vi "Variant Read.vi"   [LabVIEW 2021, in "Ring Buffer Strict Accessor Unit Tests.lvlib"]
uses:
  Ring Buffer Strict Accessor Unit Tests.lvlib
  <vilib>/Utility/Data Type/Type Definitions/Data Type.ctl
  Source/SubVIs/Endianess.ctl
  4dddbd7f-7a37-4b30-b909-1420f6624c69.vi
  9f68938b-e704-4d93-b96c-76448c5e5cfd.vi
  8e334985-5f37-4127-8ba8-a9867f1f09de.vi
  fedf0e91-6876-4bdd-8e42-2782282ca75b.vi
  21e74d2b-f5ac-4ba9-b347-dd9c42e89ba9.vi
  8a9216e5-439f-4ec4-b565-879cfa18150d.vi
  3161eb3e-d1dc-4e30-b8f9-f2ede20ab9bc.vi
  041afb3c-c61b-4d60-aacb-d153d2ee3189.vi
  26201e5a-6935-4402-8858-a5fc3b6697ee.vi
  4dddbd7f-7a37-4b30-b909-1420f6624c69.vi/4c2a6c61-f100-483c-8a49-51e57025a24c.vi
  4dddbd7f-7a37-4b30-b909-1420f6624c69.vi/e57bc314-87c7-4952-9bc8-929005dac297.vi
  <userlib>/bjustice/Ring Buffer for Time Series Data/API Poly.vi
  <userlib>/bjustice/Ring Buffer for Time Series Data/API/Write Array.vi
  9f68938b-e704-4d93-b96c-76448c5e5cfd.vi/f2df9050-0eef-46c6-aff6-3ce3a8893ea5.vi
  8e334985-5f37-4127-8ba8-a9867f1f09de.vi/17d75e1a-130a-47e0-8f2c-6c7d90b8ca77.vi
  <userlib>/bjustice/Ring Buffer for Time Series Data/API/Read Latest Value.vi
  Source/SubVIs/Index ByteArray.vi
  8e334985-5f37-4127-8ba8-a9867f1f09de.vi/19bdd28a-0674-4be3-87bb-ec701e431d75.vi
  Source/SubVIs/error if empty buffer.vi
  Source/SubVIs/ByteArray to Variant.vi
  fedf0e91-6876-4bdd-8e42-2782282ca75b.vi/4c2a6c61-f100-483c-8a49-51e57025a24c.vi
  fedf0e91-6876-4bdd-8e42-2782282ca75b.vi/e57bc314-87c7-4952-9bc8-929005dac297.vi
  21e74d2b-f5ac-4ba9-b347-dd9c42e89ba9.vi/f2df9050-0eef-46c6-aff6-3ce3a8893ea5.vi
  8a9216e5-439f-4ec4-b565-879cfa18150d.vi/17d75e1a-130a-47e0-8f2c-6c7d90b8ca77.vi
  8a9216e5-439f-4ec4-b565-879cfa18150d.vi/19bdd28a-0674-4be3-87bb-ec701e431d75.vi
  3161eb3e-d1dc-4e30-b8f9-f2ede20ab9bc.vi/4c2a6c61-f100-483c-8a49-51e57025a24c.vi
  3161eb3e-d1dc-4e30-b8f9-f2ede20ab9bc.vi/e57bc314-87c7-4952-9bc8-929005dac297.vi
  041afb3c-c61b-4d60-aacb-d153d2ee3189.vi/f2df9050-0eef-46c6-aff6-3ce3a8893ea5.vi
  26201e5a-6935-4402-8858-a5fc3b6697ee.vi/17d75e1a-130a-47e0-8f2c-6c7d90b8ca77.vi
  26201e5a-6935-4402-8858-a5fc3b6697ee.vi/19bdd28a-0674-4be3-87bb-ec701e431d75.vi
  <userlib>/bjustice/Ring Buffer for Time Series Data/SubVIs/Split Values Array.vi
  <userlib>/bjustice/Ring Buffer for Time Series Data/SubVIs/Replace Values Array Multiple Timestamps.vi
  9f68938b-e704-4d93-b96c-76448c5e5cfd.vi/f2df9050-0eef-46c6-aff6-3ce3a8893ea5.vi/63c583a5-c20f-4aba-9c90-661423dee4c4.vi
  9f68938b-e704-4d93-b96c-76448c5e5cfd.vi/f2df9050-0eef-46c6-aff6-3ce3a8893ea5.vi/52385341-3d9c-45d2-aff5-e082a4793eb1.vi
  9f68938b-e704-4d93-b96c-76448c5e5cfd.vi/f2df9050-0eef-46c6-aff6-3ce3a8893ea5.vi/37f29efa-f142-46b1-a185-f0098a95fbb6.vi
  9f68938b-e704-4d93-b96c-76448c5e5cfd.vi/f2df9050-0eef-46c6-aff6-3ce3a8893ea5.vi/84b3d231-9afe-4b6e-afae-e0be43a31e4e.vi
  9f68938b-e704-4d93-b96c-76448c5e5cfd.vi/f2df9050-0eef-46c6-aff6-3ce3a8893ea5.vi/c726271c-fc36-4bb7-8553-8945ec40c1cd.vi
  9f68938b-e704-4d93-b96c-76448c5e5cfd.vi/f2df9050-0eef-46c6-aff6-3ce3a8893ea5.vi/a7b1d944-dc88-46f5-9d3e-305d46bbe1f6.vi
  9f68938b-e704-4d93-b96c-76448c5e5cfd.vi/f2df9050-0eef-46c6-aff6-3ce3a8893ea5.vi/8abc4a6e-a1d2-4e85-879b-517e0ab55733.vi
  9f68938b-e704-4d93-b96c-76448c5e5cfd.vi/f2df9050-0eef-46c6-aff6-3ce3a8893ea5.vi/bd347357-b475-4a03-9ac5-3b85ef11aecc.vi
  9f68938b-e704-4d93-b96c-76448c5e5cfd.vi/f2df9050-0eef-46c6-aff6-3ce3a8893ea5.vi/391b36e9-a702-45e4-9499-3914f8833a58.vi
  9f68938b-e704-4d93-b96c-76448c5e5cfd.vi/f2df9050-0eef-46c6-aff6-3ce3a8893ea5.vi/44155b33-c915-49ce-9e44-a66693aa70dd.vi
  9f68938b-e704-4d93-b96c-76448c5e5cfd.vi/f2df9050-0eef-46c6-aff6-3ce3a8893ea5.vi/36977d53-dbe0-4dbc-b2ac-3dea4345b868.vi
  8e334985-5f37-4127-8ba8-a9867f1f09de.vi/17d75e1a-130a-47e0-8f2c-6c7d90b8ca77.vi/bbb64351-fa28-4ac1-b583-44e271193ecd.vi
  <userlib>/bjustice/Ring Buffer for Time Series Data/SubVIs/Newest Value Index.vi
  <userlib>/bjustice/Ring Buffer for Time Series Data/SubVIs/empty buffer check.vi
  Source/SubVIs/datatype byte size.vi
  Source/SubVIs/array sizes to number of points.vi
  8e334985-5f37-4127-8ba8-a9867f1f09de.vi/19bdd28a-0674-4be3-87bb-ec701e431d75.vi/aa0a237f-a49b-4aa2-9bbf-24aeaaef4ff4.vi
  8e334985-5f37-4127-8ba8-a9867f1f09de.vi/19bdd28a-0674-4be3-87bb-ec701e431d75.vi/f817747e-b55f-49b1-b296-570247960cc7.vi
  8e334985-5f37-4127-8ba8-a9867f1f09de.vi/19bdd28a-0674-4be3-87bb-ec701e431d75.vi/b67cd731-8231-4da5-8120-504f9e3ad781.vi
  8e334985-5f37-4127-8ba8-a9867f1f09de.vi/19bdd28a-0674-4be3-87bb-ec701e431d75.vi/a12ce15c-92b2-4055-8983-dd233974db36.vi
  8e334985-5f37-4127-8ba8-a9867f1f09de.vi/19bdd28a-0674-4be3-87bb-ec701e431d75.vi/ad0fb57a-1f12-4dd1-abc3-861d1e082269.vi
  8e334985-5f37-4127-8ba8-a9867f1f09de.vi/19bdd28a-0674-4be3-87bb-ec701e431d75.vi/ae05744d-2a39-40fb-8833-65ae5a7378b4.vi
  8e334985-5f37-4127-8ba8-a9867f1f09de.vi/19bdd28a-0674-4be3-87bb-ec701e431d75.vi/921410ec-ca2c-4978-b1f8-cfb6832fa718.vi
  8e334985-5f37-4127-8ba8-a9867f1f09de.vi/19bdd28a-0674-4be3-87bb-ec701e431d75.vi/5a029d35-35da-41f0-aa85-e6fa7c0c19bf.vi
  8e334985-5f37-4127-8ba8-a9867f1f09de.vi/19bdd28a-0674-4be3-87bb-ec701e431d75.vi/2168c955-3a02-4662-875b-0fc28cc99a83.vi
  8e334985-5f37-4127-8ba8-a9867f1f09de.vi/19bdd28a-0674-4be3-87bb-ec701e431d75.vi/523eb0df-4086-4369-b852-841bb53b1744.vi
  8e334985-5f37-4127-8ba8-a9867f1f09de.vi/19bdd28a-0674-4be3-87bb-ec701e431d75.vi/4e1502e0-4b8f-4235-a019-d1f8fa6b863c.vi
  Source/SubVIs/ByteArray to Variant.vi/8a60398d-b755-4916-b991-d3a0bc5f0417.vi
  Source/SubVIs/ByteArray to Variant.vi/751c3a01-ff04-4836-b7a6-7b574d4a9b81.vi
  Source/SubVIs/ByteArray to Variant.vi/221f450a-1b6f-46a4-a2fc-afe85f1524e2.vi
  Source/SubVIs/ByteArray to Variant.vi/41001614-cdbd-4ebb-921a-864de9ec47e2.vi
  Source/SubVIs/ByteArray to Variant.vi/5546051e-c623-4301-8272-f4bdabd7954b.vi
  Source/SubVIs/ByteArray to Variant.vi/5ca96b41-1aac-43f3-81c4-abd3cf1c6587.vi
  Source/SubVIs/ByteArray to Variant.vi/7d34a3b6-a7c4-49dd-9cdf-fb0f78c178d5.vi
  Source/SubVIs/ByteArray to Variant.vi/d8189c62-4619-451b-9af1-1c592367667c.vi
  Source/SubVIs/ByteArray to Variant.vi/ae543023-a94a-4a2d-bef6-e89c8b6f7eb3.vi
  Source/SubVIs/ByteArray to Variant.vi/788b2cc3-569e-4ae0-be57-2fef15c96938.vi
  Source/SubVIs/ByteArray to Variant.vi/2b477ad7-803c-4946-b2f4-1fc748402100.vi
  Source/SubVIs/ByteArray to Variant.vi/098c5dbb-e4d0-4c7a-81ed-dc9b4f9ca07a.vi
  Source/SubVIs/ByteArray to Variant.vi/0e7c8b9e-e897-4ed3-8864-39927aea5c8f.vi
  Source/SubVIs/ByteArray to Variant.vi/f4fc8823-9e07-4dc6-8a2a-c00e5aad4daa.vi
  Source/SubVIs/ByteArray to Variant.vi/4e00dd29-4a4f-4c51-b5d6-93aa465532c5.vi
  Source/SubVIs/ByteArray to Variant.vi/5f2f642a-ad03-4c41-b5d5-f276612f3591.vi
  Source/SubVIs/ByteArray to Variant.vi/571e8695-7815-4b46-9fe8-94e034d2cc8e.vi
  Source/SubVIs/ByteArray to Variant.vi/3d662265-0079-46bb-92db-c9b066d77669.vi
  Source/SubVIs/ByteArray to Variant.vi/817a4f5e-2c65-4066-9894-ecba4a0e477b.vi
  Source/SubVIs/ByteArray to Variant.vi/3fadb452-1f1f-455e-89f0-d18ad6ef6ba2.vi
  Source/SubVIs/ByteArray to Variant.vi/5d6b12d9-691a-45b4-9c34-a3da6780b00a.vi
  Source/SubVIs/ByteArray to Variant.vi/9891769e-6c37-4b59-a094-aa89e879cb8b.vi
  21e74d2b-f5ac-4ba9-b347-dd9c42e89ba9.vi/f2df9050-0eef-46c6-aff6-3ce3a8893ea5.vi/63c583a5-c20f-4aba-9c90-661423dee4c4.vi
  21e74d2b-f5ac-4ba9-b347-dd9c42e89ba9.vi/f2df9050-0eef-46c6-aff6-3ce3a8893ea5.vi/52385341-3d9c-45d2-aff5-e082a4793eb1.vi
  21e74d2b-f5ac-4ba9-b347-dd9c42e89ba9.vi/f2df9050-0eef-46c6-aff6-3ce3a8893ea5.vi/37f29efa-f142-46b1-a185-f0098a95fbb6.vi
  21e74d2b-f5ac-4ba9-b347-dd9c42e89ba9.vi/f2df9050-0eef-46c6-aff6-3ce3a8893ea5.vi/84b3d231-9afe-4b6e-afae-e0be43a31e4e.vi
  21e74d2b-f5ac-4ba9-b347-dd9c42e89ba9.vi/f2df9050-0eef-46c6-aff6-3ce3a8893ea5.vi/c726271c-fc36-4bb7-8553-8945ec40c1cd.vi
  21e74d2b-f5ac-4ba9-b347-dd9c42e89ba9.vi/f2df9050-0eef-46c6-aff6-3ce3a8893ea5.vi/a7b1d944-dc88-46f5-9d3e-305d46bbe1f6.vi
  21e74d2b-f5ac-4ba9-b347-dd9c42e89ba9.vi/f2df9050-0eef-46c6-aff6-3ce3a8893ea5.vi/8abc4a6e-a1d2-4e85-879b-517e0ab55733.vi
  21e74d2b-f5ac-4ba9-b347-dd9c42e89ba9.vi/f2df9050-0eef-46c6-aff6-3ce3a8893ea5.vi/bd347357-b475-4a03-9ac5-3b85ef11aecc.vi
  21e74d2b-f5ac-4ba9-b347-dd9c42e89ba9.vi/f2df9050-0eef-46c6-aff6-3ce3a8893ea5.vi/391b36e9-a702-45e4-9499-3914f8833a58.vi
  21e74d2b-f5ac-4ba9-b347-dd9c42e89ba9.vi/f2df9050-0eef-46c6-aff6-3ce3a8893ea5.vi/44155b33-c915-49ce-9e44-a66693aa70dd.vi
  21e74d2b-f5ac-4ba9-b347-dd9c42e89ba9.vi/f2df9050-0eef-46c6-aff6-3ce3a8893ea5.vi/36977d53-dbe0-4dbc-b2ac-3dea4345b868.vi
  8a9216e5-439f-4ec4-b565-879cfa18150d.vi/17d75e1a-130a-47e0-8f2c-6c7d90b8ca77.vi/bbb64351-fa28-4ac1-b583-44e271193ecd.vi
  8a9216e5-439f-4ec4-b565-879cfa18150d.vi/19bdd28a-0674-4be3-87bb-ec701e431d75.vi/81c66277-30bd-484c-9c7c-9646f36721bb.vi
  8a9216e5-439f-4ec4-b565-879cfa18150d.vi/19bdd28a-0674-4be3-87bb-ec701e431d75.vi/7ca10173-70f1-4bfb-9c4b-948090662032.vi
  8a9216e5-439f-4ec4-b565-879cfa18150d.vi/19bdd28a-0674-4be3-87bb-ec701e431d75.vi/ea4aced9-3494-4b3f-b998-02af6afbdac4.vi
  8a9216e5-439f-4ec4-b565-879cfa18150d.vi/19bdd28a-0674-4be3-87bb-ec701e431d75.vi/022c581c-5349-49df-98f9-5a038829ee63.vi
  8a9216e5-439f-4ec4-b565-879cfa18150d.vi/19bdd28a-0674-4be3-87bb-ec701e431d75.vi/ed40bcc8-bbaa-4b61-9e1a-b4b75cf21b06.vi
  8a9216e5-439f-4ec4-b565-879cfa18150d.vi/19bdd28a-0674-4be3-87bb-ec701e431d75.vi/f4b703c2-aaab-40a0-b3da-b0c22dc82d50.vi
  8a9216e5-439f-4ec4-b565-879cfa18150d.vi/19bdd28a-0674-4be3-87bb-ec701e431d75.vi/1efa054f-b143-4d96-9f7e-584a7c6fa7fd.vi
  8a9216e5-439f-4ec4-b565-879cfa18150d.vi/19bdd28a-0674-4be3-87bb-ec701e431d75.vi/b7c29f3f-256a-4401-af9d-aa15374df391.vi
  8a9216e5-439f-4ec4-b565-879cfa18150d.vi/19bdd28a-0674-4be3-87bb-ec701e431d75.vi/2fb7b479-974d-4a18-8674-c4c8d9dc9a89.vi
  8a9216e5-439f-4ec4-b565-879cfa18150d.vi/19bdd28a-0674-4be3-87bb-ec701e431d75.vi/faac7175-5814-4bb6-a961-a8db1f460653.vi
  8a9216e5-439f-4ec4-b565-879cfa18150d.vi/19bdd28a-0674-4be3-87bb-ec701e431d75.vi/b6af2a6f-71a4-4cfe-837f-b196861458b0.vi
  041afb3c-c61b-4d60-aacb-d153d2ee3189.vi/f2df9050-0eef-46c6-aff6-3ce3a8893ea5.vi/63c583a5-c20f-4aba-9c90-661423dee4c4.vi
  041afb3c-c61b-4d60-aacb-d153d2ee3189.vi/f2df9050-0eef-46c6-aff6-3ce3a8893ea5.vi/52385341-3d9c-45d2-aff5-e082a4793eb1.vi
  041afb3c-c61b-4d60-aacb-d153d2ee3189.vi/f2df9050-0eef-46c6-aff6-3ce3a8893ea5.vi/37f29efa-f142-46b1-a185-f0098a95fbb6.vi
  041afb3c-c61b-4d60-aacb-d153d2ee3189.vi/f2df9050-0eef-46c6-aff6-3ce3a8893ea5.vi/84b3d231-9afe-4b6e-afae-e0be43a31e4e.vi
  041afb3c-c61b-4d60-aacb-d153d2ee3189.vi/f2df9050-0eef-46c6-aff6-3ce3a8893ea5.vi/c726271c-fc36-4bb7-8553-8945ec40c1cd.vi
  041afb3c-c61b-4d60-aacb-d153d2ee3189.vi/f2df9050-0eef-46c6-aff6-3ce3a8893ea5.vi/a7b1d944-dc88-46f5-9d3e-305d46bbe1f6.vi
  041afb3c-c61b-4d60-aacb-d153d2ee3189.vi/f2df9050-0eef-46c6-aff6-3ce3a8893ea5.vi/8abc4a6e-a1d2-4e85-879b-517e0ab55733.vi
  041afb3c-c61b-4d60-aacb-d153d2ee3189.vi/f2df9050-0eef-46c6-aff6-3ce3a8893ea5.vi/bd347357-b475-4a03-9ac5-3b85ef11aecc.vi
  041afb3c-c61b-4d60-aacb-d153d2ee3189.vi/f2df9050-0eef-46c6-aff6-3ce3a8893ea5.vi/391b36e9-a702-45e4-9499-3914f8833a58.vi
  041afb3c-c61b-4d60-aacb-d153d2ee3189.vi/f2df9050-0eef-46c6-aff6-3ce3a8893ea5.vi/44155b33-c915-49ce-9e44-a66693aa70dd.vi
  041afb3c-c61b-4d60-aacb-d153d2ee3189.vi/f2df9050-0eef-46c6-aff6-3ce3a8893ea5.vi/36977d53-dbe0-4dbc-b2ac-3dea4345b868.vi
  26201e5a-6935-4402-8858-a5fc3b6697ee.vi/17d75e1a-130a-47e0-8f2c-6c7d90b8ca77.vi/bbb64351-fa28-4ac1-b583-44e271193ecd.vi
  26201e5a-6935-4402-8858-a5fc3b6697ee.vi/19bdd28a-0674-4be3-87bb-ec701e431d75.vi/aa0a237f-a49b-4aa2-9bbf-24aeaaef4ff4.vi
  26201e5a-6935-4402-8858-a5fc3b6697ee.vi/19bdd28a-0674-4be3-87bb-ec701e431d75.vi/f817747e-b55f-49b1-b296-570247960cc7.vi
  26201e5a-6935-4402-8858-a5fc3b6697ee.vi/19bdd28a-0674-4be3-87bb-ec701e431d75.vi/b67cd731-8231-4da5-8120-504f9e3ad781.vi
  26201e5a-6935-4402-8858-a5fc3b6697ee.vi/19bdd28a-0674-4be3-87bb-ec701e431d75.vi/a12ce15c-92b2-4055-8983-dd233974db36.vi
  26201e5a-6935-4402-8858-a5fc3b6697ee.vi/19bdd28a-0674-4be3-87bb-ec701e431d75.vi/ad0fb57a-1f12-4dd1-abc3-861d1e082269.vi
  26201e5a-6935-4402-8858-a5fc3b6697ee.vi/19bdd28a-0674-4be3-87bb-ec701e431d75.vi/ae05744d-2a39-40fb-8833-65ae5a7378b4.vi
  26201e5a-6935-4402-8858-a5fc3b6697ee.vi/19bdd28a-0674-4be3-87bb-ec701e431d75.vi/921410ec-ca2c-4978-b1f8-cfb6832fa718.vi
  26201e5a-6935-4402-8858-a5fc3b6697ee.vi/19bdd28a-0674-4be3-87bb-ec701e431d75.vi/5a029d35-35da-41f0-aa85-e6fa7c0c19bf.vi
  26201e5a-6935-4402-8858-a5fc3b6697ee.vi/19bdd28a-0674-4be3-87bb-ec701e431d75.vi/2168c955-3a02-4662-875b-0fc28cc99a83.vi
  26201e5a-6935-4402-8858-a5fc3b6697ee.vi/19bdd28a-0674-4be3-87bb-ec701e431d75.vi/523eb0df-4086-4369-b852-841bb53b1744.vi
  26201e5a-6935-4402-8858-a5fc3b6697ee.vi/19bdd28a-0674-4be3-87bb-ec701e431d75.vi/4e1502e0-4b8f-4235-a019-d1f8fa6b863c.vi
  <userlib>/bjustice/Ring Buffer for Time Series Data/SubVIs/Enforce array size multiple timestamps.vi
  Source/API/New.vi
  <vilib>/Utility/error.llb/Error Cluster From Error Code.vi
  <vilib>/Utility/error.llb/Trim Whitespace.vi
  <vilib>/addons/_JKI Toolkits/Caraya/classes/Assert/Assert Not Error.vi
  <vilib>/addons/_JKI Toolkits/Caraya/classes/Assert/Assert Equal Value_Variant.vi
  Source/Ring Buffer Strict Accessor.lvlib
  <vilib>/addons/_JKI Toolkits/Caraya/classes/Test/Test.lvclass
  <vilib>/addons/_JKI Toolkits/Caraya/classes/Assert/Assert.lvclass
  <vilib>/Utility/Data Type/NI_Data Type.lvlib
types:
  T1 = typedef "NI_Data Type.lvlib/Data Type.ctl" = enum8{"Invalid Type", "Void", "I8", "I16", "I32", "I64", "U8", "U16", "U32", "U64", "Single Float", "Double Float", "Extended Float", "Single Complex", "Double Complex", "Extended Complex", "Enum U8", "Enum U16", "Enum U32", "Enum U64", "Single Float With Unit", "Double Float With Unit", "Extended Float With Unit", "Single Complex with Unit", "Double Complex with Unit", "Extended Complex with Unit", "Boolean", "String", "Path", "Picture", "Tag", "Array", "Cluster", "Variant", "LV Variant", "Waveform", "Timestamp", "Digital Waveform", "Digital Data", "ExpressData", "Refnum", "External Data", "VI", "Poly VI", "LabVIEW Class Instance", "Fixed Point", "Set Collection", "Map Collection"}
  T2 = typedef "Ring Buffer Strict Accessor.lvlib/Endianess.ctl" = enum16{"big-endian", "little-endian"}
  T3 = typedef "Ring Buffer Strict Accessor.lvlib/RingBufferHandle.ctl" = cluster{"Ring buffer DVR":refnum<data-value>, "Data Type":T4, "Size(s)":i32[], "Endianess":T2, "Buffer Size (#timestamps) [init]":i32}
  T4 = typedef "Ring Buffer Strict Accessor.lvlib/DataType.ctl" = enum16{"uint8", "uint16", "uint32", "uint64", "int8", "int16", "int32", "int64", "float", "double", "extended"}
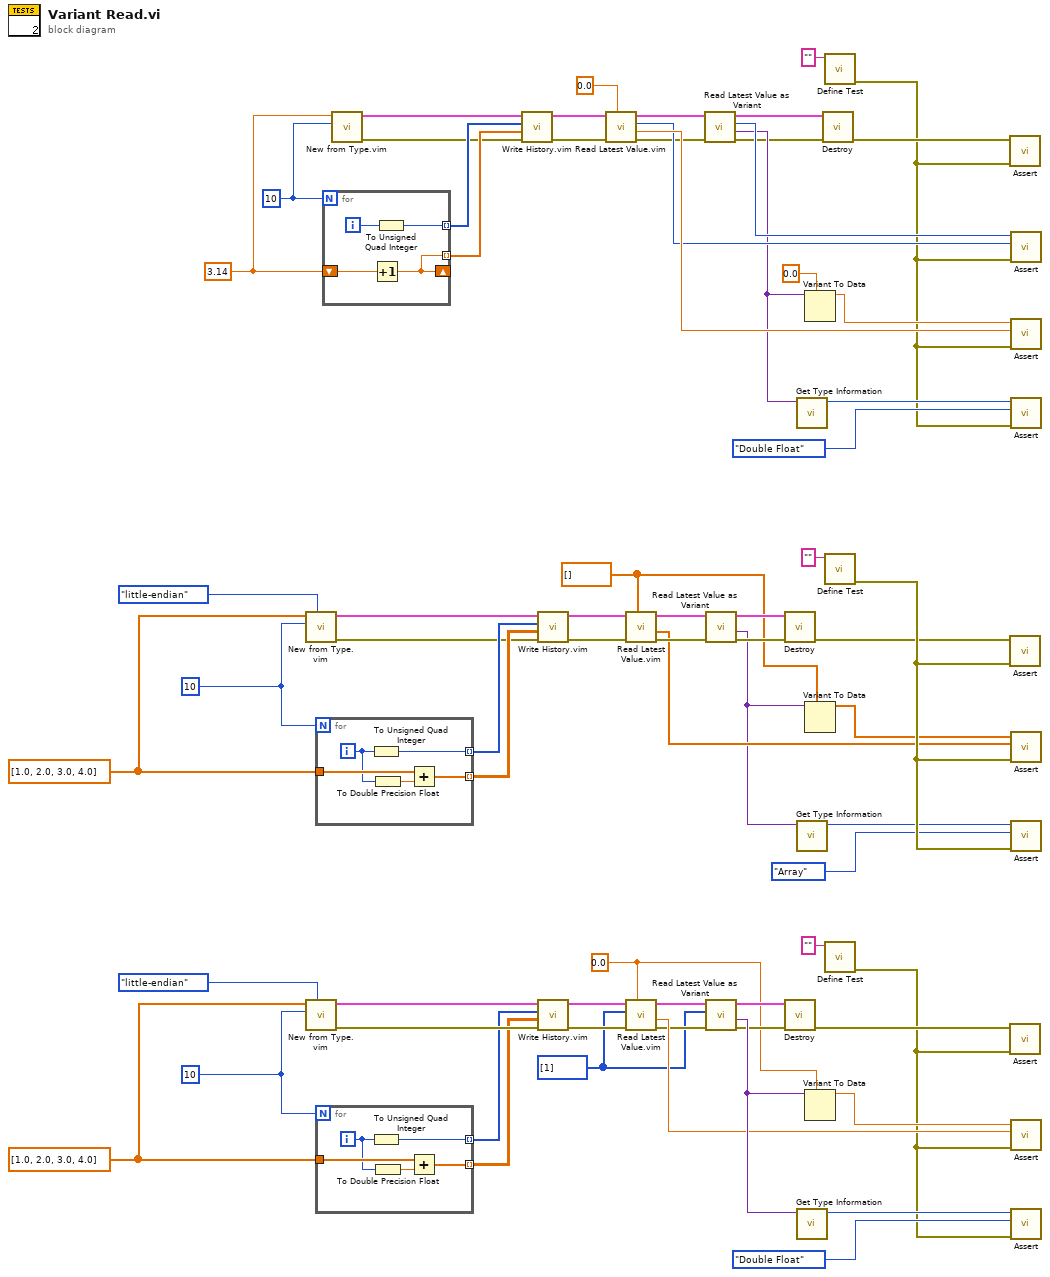
[diagram p0: block diagram]
diagram:
  w3 = i32[] [1] ("index")
  w2 = 0.0
  w10 = 10 ("Buffer Size (#timestamps)")
  w9 = dbl[] [1.0, 2.0, 3.0, 4.0]
  w1 = dbl[] []
  w39 = 10 ("Buffer Size (#timestamps)")
  w40 = dbl[] [1.0, 2.0, 3.0, 4.0]
  w67 = 10 ("Buffer Size (#timestamps)")
  w69 = 3.14 ("LV type")
  n1 = call "New from Type.vim"("Endianess"=Endianess."little-endian", "Buffer Size (#timestamps)"=w39, "LV type (array size cannot be empty)"=w40) -> ("error out"=w41:errorcluster, "Ring Buffer"=w42:T3)  [unwired: 7 in]
  n2 = call "New from Type.vim"("Endianess"=Endianess."little-endian", "Buffer Size (#timestamps)"=w10, "LV type (array size cannot be empty)"=w9) -> ("error out"=w8:errorcluster, "Ring Buffer"=w7:T3)  [unwired: 7 in]
  n3 = for {
    N: w39 -> [_]
    tunnel: w40 -> [w74]
    tunnel: [w73] -> w44 mode=indexing
    tunnel: [w72] -> w45 mode=indexing
    i -> [w71]
    n4 = To Unsigned Quad Integer(1:w71) -> (0:w72:u64)
    n5 = To Double Precision Float(number=w71) -> (double precision float=w70:dbl)
    n6 = Add(x=w74, y=w70) -> (x+y=w73:dbl[])
  }
  n7 = for {
    N: w10 -> [_]
    tunnel: w9 -> [w79]
    tunnel: [w78] -> w5 mode=indexing
    tunnel: [w77] -> w4 mode=indexing
    i -> [w76]
    n8 = To Unsigned Quad Integer(1:w76) -> (0:w77:u64)
    n9 = To Double Precision Float(number=w76) -> (double precision float=w75:dbl)
    n10 = Add(x=w79, y=w75) -> (x+y=w78:dbl[])
  }
  n11 = for {
    N: w67 -> [_]
    tunnel: [w81] -> w66 mode=indexing
    shift-right: [w80] -> _
    shift-left: w69 -> [w82]
    tunnel: [w80] -> w65 mode=indexing
    i -> [w83]
    n12 = Increment(x=w82) -> (x+1=w80:dbl)
    n13 = To Unsigned Quad Integer(1:w83) -> (0:w81:u64)
  }
  n14 = call "New from Type.vim"("Buffer Size (#timestamps)"=w67, "LV type (array size cannot be empty)"=w69) -> ("error out"=w52:errorcluster, "Ring Buffer"=w68:T3)  [unwired: 8 in]
  n15 = call "Write History.vim"("error in (no error)"=w52, "LV DataType"=w65, "Timestamps"=w66, "Ring Buffer"=w68) -> ("error out"=w51:errorcluster, "Ring Buffer"=w62:T3)  [unwired: 6 in]
  n16 = call "Write History.vim"("error in (no error)"=w41, "LV DataType"=w44, "Timestamps"=w45, "Ring Buffer"=w42) -> ("error out"=w37:errorcluster, "Ring Buffer"=w38:T3)  [unwired: 6 in]
  n17 = call "Write History.vim"("error in (no error)"=w8, "LV DataType"=w5, "Timestamps"=w4, "Ring Buffer"=w7) -> ("error out"=w12:errorcluster, "Ring Buffer"=w11:T3)  [unwired: 6 in]
  n18 = call "Read Latest Value.vim"("data type"=0.0 ("LV type"), "error in (no error)"=w51, "Ring Buffer"=w62) -> ("error out"=w50:errorcluster, "Values"=w58:dbl, "Timestamps"=w56:u64, "Ring Buffer"=w64:T3)  [unwired: 5 in]
  n19 = call "Read Latest Value.vim"("data type"=w1, "error in (no error)"=w37, "Ring Buffer"=w38) -> ("error out"=w35:errorcluster, "Values"=w26:dbl[], "Ring Buffer"=w36:T3)  [unwired: 5 in, 1 out]
  n20 = call "Read Latest Value.vim"("data type"=w2, "error in (no error)"=w12, "index"=w3, "Ring Buffer"=w11) -> ("error out"=w14:errorcluster, "Values"=w23:dbl, "Ring Buffer"=w13:T3)  [unwired: 4 in, 1 out]
  n21 = call "Read Latest Value as Variant.vi"("error in (no error)"=w50, "Ring Buffer"=w64) -> ("error out"=w49:errorcluster, "Values"=w55:variant, "Timestamps"=w57:u64, "Ring Buffer"=w63:T3)  [unwired: 6 in]
  n22 = call "Read Latest Value as Variant.vi"("error in (no error)"=w35, "Ring Buffer"=w36) -> ("error out"=w33:errorcluster, "Values"=w25:variant, "Ring Buffer"=w34:T3)  [unwired: 6 in, 1 out]
  n23 = call "Read Latest Value as Variant.vi"("error in (no error)"=w14, "index"=w3, "Ring Buffer"=w13) -> ("error out"=w16:errorcluster, "Values"=w24:variant, "Ring Buffer"=w15:T3)  [unwired: 5 in, 1 out]
  n24 = call "Destroy.vi"("error in (no error)"=w33, "Ring Buffer"=w34) -> ("error out"=w28:errorcluster)  [unwired: 9 in]
  n25 = call "Destroy.vi"("error in (no error)"=w16, "Ring Buffer"=w15) -> ("error out"=w21:errorcluster)  [unwired: 9 in]
  n26 = call <vilib>:"Get Type Information.vi"("variant"=w55) -> ("type"=w54:T1)  [unwired: 6 in, 4 out]
  n27 = call <vilib>:"Get Type Information.vi"("variant"=w25) -> ("type"=w30:T1)  [unwired: 6 in, 4 out]
  n28 = call <vilib>:"Get Type Information.vi"("variant"=w24) -> ("type"=w19:T1)  [unwired: 6 in, 4 out]
  n29 = Variant To Data(type=0.0 ("LV type"), Variant=w55) -> (data=w59:dbl)  [unwired: 1 in, 1 out]
  n30 = Variant To Data(type=w1, Variant=w25) -> (data=w27:dbl[])  [unwired: 1 in, 1 out]
  n31 = Variant To Data(type=w2, Variant=w24) -> (data=w22:dbl)  [unwired: 1 in, 1 out]
  n32 = call "Destroy.vi"("error in (no error)"=w49, "Ring Buffer"=w63) -> ("error out"=w48:errorcluster)  [unwired: 9 in]
  n33 = call <vilib>:"Define Test.vi"("Label (VI Title)"="") -> ("error out"=w47:errorcluster)  [unwired: 9 in, 1 out]
  n34 = call <vilib>:"Define Test.vi"("Label (VI Title)"="") -> ("error out"=w32:errorcluster)  [unwired: 9 in, 1 out]
  n35 = call <vilib>:"Define Test.vi"("Label (VI Title)"="") -> ("error out"=w17:errorcluster)  [unwired: 9 in, 1 out]
  n36 = call-poly <vilib>:"Assert.vi"("error in (no error)"=w47, "Not Error?"=w48) -> ()  [unwired: 8 in, 2 out]
  n37 = call-poly <vilib>:"Assert.vi"("error in (no error)"=w32, "Not Error?"=w28) -> ()  [unwired: 8 in, 2 out]
  n38 = call-poly <vilib>:"Assert.vi"("error in (no error)"=w17, "Not Error?"=w21) -> ()  [unwired: 8 in, 2 out]
  n39 = call-poly <vilib>:"Assert.vi"("error in (no error)"=w47, "Y"=w56, "X"=w57) -> ()  [unwired: 7 in, 2 out]
  n40 = call-poly <vilib>:"Assert.vi"("error in (no error)"=w47, "Y"=w58, "X"=w59) -> ()  [unwired: 7 in, 2 out]
  n41 = call-poly <vilib>:"Assert.vi"("error in (no error)"=w47, "Y"=Data_Type."Double Float" ("type"), "X"=w54) -> ()  [unwired: 7 in, 2 out]
  n42 = call-poly <vilib>:"Assert.vi"("error in (no error)"=w32, "Y"=w26, "X"=w27) -> ()  [unwired: 7 in, 2 out]
  n43 = call-poly <vilib>:"Assert.vi"("error in (no error)"=w32, "Y"=Data_Type."Array" ("type"), "X"=w30) -> ()  [unwired: 7 in, 2 out]
  n44 = call-poly <vilib>:"Assert.vi"("error in (no error)"=w17, "Y"=w23, "X"=w22) -> ()  [unwired: 7 in, 2 out]
  n45 = call-poly <vilib>:"Assert.vi"("error in (no error)"=w17, "Y"=Data_Type."Double Float" ("type"), "X"=w19) -> ()  [unwired: 7 in, 2 out]
